vi "Dresden R2R Sputter 03.02.2018 IY24.vi"() -> ()   [LabVIEW 2009] (continued)
                      n14016 = case shown="False" w20577 {
                        tunnel: [FALSE ("Casette_servo_left_direction_do") TRUE ("Casette_servo_left_direction_do")] -> w20576
                        frame #0 {
                          n14017 = Wait Until Next ms Multiple(millisecond multiple=u32 200) -> ()  [unwired: 1 out]
                          n14018 = local write "Casette_servo_start/stop_do"(TRUE ("Casette_servo_left_direction_do")) -> ()
                        }
                        frame #1 {
                        }
                      }
                      n14019 = local read "Semi"() -> (w20575:bool)
                      n14020 = Or(x=w20576, y=w20575) -> (x .or. y?=w20574:bool)
                    }
                  }
                  frame #1 {
                    n14021 = local read "Semi"() -> (w20587:bool)
                    n14022 = case shown="False" w20587 {
                      frame #0 {
                        n14023 = local write "CH1_2trns_11"(TRUE ("CH1_2trns_9")) -> ()
                        n14024 = Wait (ms)(milliseconds to wait=u32 500) -> ()  [unwired: 1 out]
                      }
                      frame #1 {
                      }
                    }
                  }
                }
              }
              frame #1 {
              }
            }
          }
          frame #16 {
            # "Left sensors activate"
            n14025 = local read "Semi"() -> (w20590:bool)
            n14026 = case shown="False" w20590 {
              frame #0 {
                n14027 = stacked-sequence {
                  frame #0 {
                    n14028 = while {
                      i -> [w20599]
                      stop <- w20595 stop-if-true
                      n14029 = local read "Counter_read_data"() -> (w20592:i16)
                      n14030 = Greater?(x=w20599, y=1500) -> (0:w20598:bool)
                      n14031 = case shown="True" w20598 {
                        frame #0 {
                        }
                        frame #1 {
                          n14032 = local write "Semi"(TRUE ("Semi")) -> ()
                          n14033 = local write "Error Message"("Transfer process was cancelled.\nPlease check Casette & Sensor\nconnections." ("Error Message")) -> ()
                        }
                      }
                      n14034 = Greater Or Equal?(x=w20592, y=i16 5800) -> (x >= y?=w20593:bool)
                      n14035 = case shown="False" w20593 {
                        tunnel: [FALSE TRUE] -> w20596
                        frame #0 {
                          n14036 = Wait Until Next ms Multiple(millisecond multiple=u32 200) -> ()  [unwired: 1 out]
                        }
                        frame #1 {
                        }
                      }
                      n14037 = local read "Semi"() -> (w20594:bool)
                      n14038 = Or(x=w20596, y=w20594) -> (x .or. y?=w20595:bool)
                    }
                  }
                  frame #1 {
                    n14039 = while {
                      i -> [w20608]
                      stop <- w20605 stop-if-true
                      n14040 = Greater?(x=w20608, y=50) -> (0:w20609:bool)
                      n14041 = local read "Cnt_Left_slow_di"() -> (w20611:bool)
                      n14042 = case shown="True" w20609 {
                        frame #0 {
                        }
                        frame #1 {
                          n14043 = local write "Semi"(TRUE ("Semi")) -> ()
                          n14044 = local write "Error Message"("\nPlease check Left Slow Sensor\nconnections." ("Error Message")) -> ()
                        }
                      }
                      n14045 = case shown="True" w20611 {
                        tunnel: [TRUE ("Cnt_Left_slow_do") FALSE ("Cnt_Left_slow_do")] -> w20607
                        frame #0 {
                        }
                        frame #1 {
                          n14046 = Wait Until Next ms Multiple(millisecond multiple=u32 200) -> ()  [unwired: 1 out]
                          n14047 = local write "Cnt_Left_slow_do"(FALSE ("Cnt_Left_slow_do")) -> ()
                        }
                      }
                      n14048 = local read "Semi"() -> (w20606:bool)
                      n14049 = Or(x=w20607, y=w20606) -> (x .or. y?=w20605:bool)
                    }
                  }
                  frame #2 {
                    n14050 = while {
                      i -> [w20621]
                      stop <- w20618 stop-if-true
                      n14051 = Greater?(x=w20621, y=50) -> (0:w20622:bool)
                      n14052 = local read "Cnt_Left_limit_di"() -> (w20624:bool)
                      n14053 = case shown="True" w20622 {
                        frame #0 {
                        }
                        frame #1 {
                          n14054 = local write "Semi"(TRUE ("Semi")) -> ()
                          n14055 = local write "Error Message"("\nPlease check Left Limit Sensor\n connections." ("Error Message")) -> ()
                        }
                      }
                      n14056 = case shown="False" w20624 {
                        tunnel: [TRUE ("Cnt_Left_slow_do") FALSE ("Cnt_Left_slow_do")] -> w20620
                        frame #0 {
                        }
                        frame #1 {
                          n14057 = Wait Until Next ms Multiple(millisecond multiple=u32 200) -> ()  [unwired: 1 out]
                          n14058 = local write "Cnt_Left_limit_do"(FALSE ("Cnt_Left_slow_do")) -> ()
                        }
                      }
                      n14059 = local read "Semi"() -> (w20619:bool)
                      n14060 = Or(x=w20620, y=w20619) -> (x .or. y?=w20618:bool)
                    }
                  }
                  frame #3 {
                    n14061 = local read "Semi"() -> (w20631:bool)
                    n14062 = case shown="False" w20631 {
                      frame #0 {
                        n14063 = local write "CH1_2trns_12"(TRUE ("CH1_2trns_11")) -> ()
                        n14064 = Wait (ms)(milliseconds to wait=u32 500) -> ()  [unwired: 1 out]
                      }
                      frame #1 {
                      }
                    }
                  }
                }
              }
              frame #1 {
              }
            }
          }
          frame #17 {
            # "SET CASSETTE SERVO  SPEED 100"
            n14065 = local read "Semi"() -> (w20634:bool)
            n14066 = case shown="False" w20634 {
              frame #0 {
                n14067 = stacked-sequence {
                  frame #0 {
                    n14068 = while {
                      i -> [w20641]
                      stop <- w20637 stop-if-true
                      n14069 = local read "Ch4_Left_slow_di"() -> (w20635:bool)
                      n14070 = Greater?(x=w20641, y=1500) -> (0:w20640:bool)
                      n14071 = case shown="True" w20640 {
                        frame #0 {
                        }
                        frame #1 {
                          n14072 = local write "Semi"(TRUE ("Semi")) -> ()
                          n14073 = local write "Error Message"("Transfer process was cancelled.\nPlease check Casette & Sensor\nconnections." ("Error Message")) -> ()
                        }
                      }
                      n14074 = case shown="True" w20635 {
                        tunnel: [FALSE TRUE] -> w20638
                        frame #0 {
                          n14075 = Wait Until Next ms Multiple(millisecond multiple=u32 200) -> ()  [unwired: 1 out]
                        }
                        frame #1 {
                        }
                      }
                      n14076 = local read "Semi"() -> (w20636:bool)
                      n14077 = Or(x=w20638, y=w20636) -> (x .or. y?=w20637:bool)
                    }
                  }
                  frame #1 {
                    n14078 = disable-structure shown="Disabled" {
                      frame #0 {
                        n14079 = while {
                          i -> [w20656]
                          stop <- w20652 stop-if-true
                          n14080 = local read "Counter_read_data"() -> (w20649:i16)
                          n14081 = Greater?(x=w20656, y=5000) -> (0:w20655:bool)
                          n14082 = case shown="True" w20655 {
                            frame #0 {
                            }
                            frame #1 {
                              n14083 = local write "Semi"(TRUE ("Semi")) -> ()
                            }
                          }
                          n14084 = In Range and Coerce(upper limit=i16 1990, x=w20649, lower limit=i16 1980 ("upper limit")) -> (In Range?=w20647:bool)  [unwired: 1 out]
                          n14085 = case shown="True" w20647 {
                            tunnel: [FALSE TRUE] -> w20653
                            frame #0 {
                              n14086 = Wait Until Next ms Multiple(millisecond multiple=u32 200) -> ()  [unwired: 1 out]
                            }
                            frame #1 {
                            }
                          }
                          n14087 = local read "Semi"() -> (w20651:bool)
                          n14088 = Or(x=w20653, y=w20651) -> (x .or. y?=w20652:bool)
                        }
                      }
                      frame #1 {
                      }
                    }
                  }
                  frame #2 {
                    n14089 = local read "Semi"() -> (w20661:bool)
                    n14090 = case shown="False" w20661 {
                      frame #0 {
                        n14091 = local write "Cassette_servo_speed_value"(u16 100 ("Cassette_servo_speed_value")) -> ()
                      }
                      frame #1 {
                      }
                    }
                  }
                  frame #3 {
                    n14092 = local read "Semi"() -> (w20663:bool)
                    n14093 = case shown="False" w20663 {
                      frame #0 {
                        n14094 = Wait (ms)(milliseconds to wait=u32 200 ("millisecond multiple")) -> ()  [unwired: 1 out]
                      }
                      frame #1 {
                      }
                    }
                  }
                  frame #4 {
                    n14095 = local read "Semi"() -> (w20665:bool)
                    n14096 = case shown="False" w20665 {
                      frame #0 {
                        n14097 = local write "Cassette_servo_speed_auto_set"(TRUE ("Cassette_servo_speed_auto_set")) -> ()
                      }
                      frame #1 {
                      }
                    }
                  }
                  frame #5 {
                    n14098 = local read "Semi"() -> (w20667:bool)
                    n14099 = case shown="False" w20667 {
                      frame #0 {
                        n14100 = Wait (ms)(milliseconds to wait=u32 200 ("millisecond multiple")) -> ()  [unwired: 1 out]
                      }
                      frame #1 {
                      }
                    }
                  }
                  frame #6 {
                    n14101 = while {
                      i -> [w20672]
                      stop <- w20669 stop-if-true
                      n14102 = Greater?(x=w20672, y=50) -> (0:w20673:bool)
                      n14103 = local read "Cnt_Left_slow_di"() -> (w20675:bool)
                      n14104 = case shown="True" w20673 {
                        frame #0 {
                        }
                        frame #1 {
                          n14105 = local write "Semi"(TRUE ("Semi")) -> ()
                          n14106 = local write "Error Message"("\nPlease check connections." ("Error Message")) -> ()
                        }
                      }
                      n14107 = case shown="False" w20675 {
                        tunnel: [FALSE ("Cnt_Left_slow_do") TRUE ("Cnt_Left_slow_do")] -> w20671
                        frame #0 {
                          n14108 = Wait Until Next ms Multiple(millisecond multiple=u32 200) -> ()  [unwired: 1 out]
                          n14109 = local write "Cnt_Left_slow_do"(TRUE ("Cnt_Left_slow_do")) -> ()
                        }
                        frame #1 {
                        }
                      }
                      n14110 = local read "Semi"() -> (w20670:bool)
                      n14111 = Or(x=w20671, y=w20670) -> (x .or. y?=w20669:bool)
                    }
                  }
                  frame #7 {
                    n14112 = local read "Semi"() -> (w20682:bool)
                    n14113 = case shown="False" w20682 {
                      frame #0 {
                        n14114 = local write "CH1_2trns_12"(TRUE ("CH1_2trns_11")) -> ()
                        n14115 = Wait (ms)(milliseconds to wait=u32 500) -> ()  [unwired: 1 out]
                      }
                      frame #1 {
                      }
                    }
                  }
                }
              }
              frame #1 {
              }
            }
          }
          frame #18 {
            # "CASETTE STOP AND FIX"
            n14116 = local read "Semi"() -> (w20685:bool)
            n14117 = case shown="False" w20685 {
              frame #0 {
                n14118 = stacked-sequence {
                  frame #0 {
                    # "Center Casette stop"
                    n14119 = local read "Semi"() -> (w20686:bool)
                    n14120 = case shown="False" w20686 {
                      frame #0 {
                        n14121 = stacked-sequence {
                          frame #0 {
                            n14122 = while {
                              i -> [w20693]
                              stop <- w20688 stop-if-true
                              n14123 = local read "Ch4_Left_limit_di"() -> (w20687:bool)
                              n14124 = Greater?(x=w20693, y=600) -> (0:w20691:bool)
                              n14125 = case shown="True" w20691 {
                                frame #0 {
                                }
                                frame #1 {
                                n14126 = local write "Semi"(TRUE ("Semi")) -> ()
                                n14127 = local write "Error Message"("Transfer process was cancelled.\nPlease check Casette connections." ("Error Message")) -> ()
                                }
                              }
                              n14128 = case shown="False" w20687 {
                                tunnel: [FALSE TRUE] -> w20690
                                frame #0 {
                                n14129 = Wait Until Next ms Multiple(millisecond multiple=u32 200) -> ()  [unwired: 1 out]
                                }
                                frame #1 {
                                }
                              }
                              n14130 = local read "Semi"() -> (w20689:bool)
                              n14131 = Or(x=w20690, y=w20689) -> (x .or. y?=w20688:bool)
                            }
                          }
                          frame #1 {
                            n14132 = disable-structure shown="Disabled" {
                              frame #0 {
                                n14133 = while {
                                i -> [w20708]
                                stop <- w20703 stop-if-true
                                n14134 = local read "Counter_read_data"() -> (w20700:i16)
                                n14135 = Greater?(x=w20708, y=5000) -> (0:w20706:bool)
                                n14136 = case shown="True" w20706 {
                                frame #0 {
                                }
                                frame #1 {
                                n14137 = local write "Semi"(TRUE ("Semi")) -> ()
                                n14138 = local write "Error Message"("Transfer process was cancelled.\nPlease check Casette connections." ("Error Message")) -> ()
                                }
                                }
                                n14139 = In Range and Coerce(upper limit=i16 2209, x=w20700, lower limit=i16 2199 ("upper limit")) -> (In Range?=w20699:bool)  [unwired: 1 out]
                                n14140 = case shown="True" w20699 {
                                tunnel: [FALSE TRUE] -> w20705
                                frame #0 {
                                }
                                frame #1 {
                                n14141 = Wait Until Next ms Multiple(millisecond multiple=u32 500) -> ()  [unwired: 1 out]
                                }
                                }
                                n14142 = local read "Semi"() -> (w20704:bool)
                                n14143 = Or(x=w20705, y=w20704) -> (x .or. y?=w20703:bool)
                                }
                              }
                              frame #1 {
                              }
                            }
                          }
                          frame #2 {
                            n14144 = while {
                              i -> [w20720]
                              stop <- w20715 stop-if-true
                              n14145 = local read "Casette_servo_start/stop_di"() -> (w20714:bool)
                              n14146 = Greater?(x=w20720, y=50) -> (0:w20718:bool)
                              n14147 = case shown="True" w20718 {
                                frame #0 {
                                }
                                frame #1 {
                                n14148 = local write "Semi"(TRUE ("Semi")) -> ()
                                n14149 = local write "Error Message"("Transfer process was cancelled.\nPlease check Casette connections." ("Error Message")) -> ()
                                }
                              }
                              n14150 = case shown="True" w20714 {
                                tunnel: [TRUE FALSE] -> w20717
                                frame #0 {
                                }
                                frame #1 {
                                n14151 = Wait Until Next ms Multiple(millisecond multiple=u32 200) -> ()  [unwired: 1 out]
                                n14152 = local write "Casette_servo_start/stop_do"(FALSE ("Casette_servo_start/stop_di")) -> ()
                                }
                              }
                              n14153 = local read "Semi"() -> (w20716:bool)
                              n14154 = Or(x=w20717, y=w20716) -> (x .or. y?=w20715:bool)
                            }
                          }
                          frame #3 {
                            n14155 = local read "Semi"() -> (w20727:bool)
                            n14156 = case shown="False" w20727 {
                              frame #0 {
                                n14157 = Wait (ms)(milliseconds to wait=u32 200) -> ()  [unwired: 1 out]
                              }
                              frame #1 {
                              }
                            }
                          }
                          frame #4 {
                            n14158 = local read "Semi"() -> (w20729:bool)
                            n14159 = case shown="False" w20729 {
                              frame #0 {
                                n14160 = local write "Cassette_servo_speed_value"(u16 0 ("Cassette_servo_speed_value")) -> ()
                              }
                              frame #1 {
                              }
                            }
                          }
                          frame #5 {
                            n14161 = local read "Semi"() -> (w20731:bool)
                            n14162 = case shown="False" w20731 {
                              frame #0 {
                                n14163 = Wait (ms)(milliseconds to wait=u32 200) -> ()  [unwired: 1 out]
                              }
                              frame #1 {
                              }
                            }
                          }
                          frame #6 {
                            n14164 = local read "Semi"() -> (w20733:bool)
                            n14165 = case shown="False" w20733 {
                              frame #0 {
                                n14166 = local write "Cassette_servo_speed_auto_set"(TRUE ("Cassette_servo_speed_auto_set")) -> ()
                              }
                              frame #1 {
                              }
                            }
                          }
                          frame #7 {
                            n14167 = local read "Semi"() -> (w20735:bool)
                            n14168 = case shown="False" w20735 {
                              frame #0 {
                                n14169 = Wait (ms)(milliseconds to wait=u32 200) -> ()  [unwired: 1 out]
                              }
                              frame #1 {
                              }
                            }
                          }
                          frame #8 {
                            n14170 = local read "Semi"() -> (w20737:bool)
                            n14171 = case shown="False" w20737 {
                              frame #0 {
                                n14172 = local write "CH1_2trns_13"(TRUE ("CH1_2trns_9")) -> ()
                                n14173 = Wait (ms)(milliseconds to wait=u32 500) -> ()  [unwired: 1 out]
                              }
                              frame #1 {
                              }
                            }
                          }
                        }
                      }
                      frame #1 {
                      }
                    }
                  }
                  frame #1 {
                    # "CASETTE FIX DOWN CH2"
                    n14174 = local read "Semi"() -> (w20740:bool)
                    n14175 = case shown="False" w20740 {
                      frame #0 {
                        n14176 = stacked-sequence {
                          frame #0 {
                            n14177 = local read "Semi"() -> (w20741:bool)
                            n14178 = case shown="False" w20741 {
                              frame #0 {
                                n14179 = while {
                                i -> [w20748]
                                stop <- w20743 stop-if-true
                                n14180 = Greater?(x=w20748, y=50) -> (0:w20746:bool)
                                n14181 = local read "Ch4_Cst_fix_down_di"() -> (w20742:bool)
                                n14182 = case shown="True" w20746 {
                                frame #0 {
                                }
                                frame #1 {
                                n14183 = local write "Semi"(TRUE ("Semi")) -> ()
                                n14184 = local write "Error Message"("Up/Down positions could not reach\nthe down position.\nPlease check connections." ("Error Message")) -> ()
                                }
                                }
                                n14185 = case shown="False" w20742 {
                                tunnel: [FALSE TRUE] -> w20745
                                frame #0 {
                                n14186 = Wait Until Next ms Multiple(millisecond multiple=u32 200) -> ()  [unwired: 1 out]
                                n14187 = local write "Ch4_Cst_fix_do"(TRUE ("Ch1_pet_cool_up_do")) -> ()
                                }
                                frame #1 {
                                }
                                }
                                n14188 = local read "Semi"() -> (w20744:bool)
                                n14189 = Or(x=w20745, y=w20744) -> (x .or. y?=w20743:bool)
                                }
                              }
                              frame #1 {
                              }
                            }
                          }
                          frame #1 {
                            n14190 = local read "Semi"() -> (w20755:bool)
                            n14191 = case shown="False" w20755 {
                              frame #0 {
                                n14192 = local write "CH1_2trns_14"(TRUE ("CH1_2trns_9")) -> ()
                                n14193 = Wait (ms)(milliseconds to wait=u32 500) -> ()  [unwired: 1 out]
                              }
                              frame #1 {
                              }
                            }
                          }
                        }
                      }
                      frame #1 {
                      }
                    }
                  }
                  frame #2 {
                    n14194 = local read "Semi"() -> (w20758:bool)
                    n14195 = case shown="False" w20758 {
                      frame #0 {
                        n14196 = stacked-sequence {
                          frame #0 {
                            n14197 = local read "Semi"() -> (w20759:bool)
                            n14198 = case shown="False" w20759 {
                              frame #0 {
                                n14199 = while {
                                i -> [w20766]
                                stop <- w20761 stop-if-true
                                n14200 = Greater?(x=w20766, y=50) -> (0:w20764:bool)
                                n14201 = local read "Ch4_Trns_gv_bp_di"() -> (w20760:bool)
                                n14202 = case shown="True" w20764 {
                                frame #0 {
                                }
                                frame #1 {
                                n14203 = local write "Semi"(TRUE ("Semi")) -> ()
                                n14204 = local write "Error Message"("Transfer process was cancelled.\nPlease check CH1-Trns-GV connections." ("Error Message")) -> ()
                                }
                                }
                                n14205 = case shown="True" w20760 {
                                tunnel: [TRUE FALSE] -> w20763
                                frame #0 {
                                }
                                frame #1 {
                                n14206 = Wait Until Next ms Multiple(millisecond multiple=u32 200) -> ()  [unwired: 1 out]
                                n14207 = local write "Ch4_Trns_gv_bp_do"(FALSE ("Ch1_pet_cool_up_do")) -> ()
                                }
                                }
                                n14208 = local read "Semi"() -> (w20762:bool)
                                n14209 = Or(x=w20763, y=w20762) -> (x .or. y?=w20761:bool)
                                }
                              }
                              frame #1 {
                              }
                            }
                          }
                          frame #1 {
                            n14210 = local read "Semi"() -> (w20773:bool)
                            n14211 = case shown="False" w20773 {
                              frame #0 {
                                n14212 = Wait (ms)(milliseconds to wait=u32 500) -> ()  [unwired: 1 out]
                              }
                              frame #1 {
                              }
                            }
                          }
                          frame #2 {
                            n14213 = local read "Semi"() -> (w20775:bool)
                            n14214 = case shown="False" w20775 {
                              frame #0 {
                                n14215 = while {
                                i -> [w20782]
                                stop <- w20777 stop-if-true
                                n14216 = Greater?(x=w20782, y=50) -> (0:w20780:bool)
                                n14217 = local read "Ch3_Trns_gv_bp2_di"() -> (w20776:bool)
                                n14218 = case shown="True" w20780 {
                                frame #0 {
                                }
                                frame #1 {
                                n14219 = local write "Semi"(TRUE ("Semi")) -> ()
                                n14220 = local write "Error Message"("Transfer process was cancelled.\nPlease check CH1-Trns-GV connections." ("Error Message")) -> ()
                                }
                                }
                                n14221 = case shown="True" w20776 {
                                tunnel: [TRUE FALSE] -> w20779
                                frame #0 {
                                }
                                frame #1 {
                                n14222 = local write "Ch3_Trns_gv_bp2_do"(FALSE ("Ch1_pet_cool_up_do")) -> ()
                                n14223 = Wait Until Next ms Multiple(millisecond multiple=u32 200) -> ()  [unwired: 1 out]
                                }
                                }
                                n14224 = local read "Semi"() -> (w20778:bool)
                                n14225 = Or(x=w20779, y=w20778) -> (x .or. y?=w20777:bool)
                                }
                              }
                              frame #1 {
                              }
                            }
                          }
                          frame #3 {
                            n14226 = local read "Semi"() -> (w20789:bool)
                            n14227 = case shown="False" w20789 {
                              frame #0 {
                                n14228 = Wait (ms)(milliseconds to wait=u32 500) -> ()  [unwired: 1 out]
                              }
                              frame #1 {
                              }
                            }
                          }
                        }
                      }
                      frame #1 {
                      }
                    }
                  }
                  frame #3 {
                    n14229 = local read "Semi"() -> (w20791:bool)
                    n14230 = case shown="False" w20791 {
                      frame #0 {
                        n14231 = stacked-sequence {
                          frame #0 {
                            n14232 = local read "Semi"() -> (w20792:bool)
                            n14233 = case shown="False" w20792 {
                              frame #0 {
                                n14234 = local write "Ch3_Trns_gv_open_do"(FALSE ("Ch1_pet_cool_up_do")) -> ()
                              }
                              frame #1 {
                              }
                            }
                          }
                          frame #1 {
                            n14235 = local read "Semi"() -> (w20794:bool)
                            n14236 = case shown="False" w20794 {
                              frame #0 {
                                n14237 = while {
                                i -> [w20801]
                                stop <- w20796 stop-if-true
                                n14238 = Greater?(x=w20801, y=500) -> (0:w20799:bool)
                                n14239 = local read "Ch3_Trns_gv_close_di"() -> (w20795:bool)
                                n14240 = case shown="True" w20799 {
                                frame #0 {
                                }
                                frame #1 {
                                n14241 = local write "Semi"(TRUE ("Semi")) -> ()
                                n14242 = local write "Error Message"("Transfer process was cancelled.\nPlease check  GV connections." ("Error Message")) -> ()
                                }
                                }
                                n14243 = case shown="False" w20795 {
                                tunnel: [FALSE TRUE] -> w20798
                                frame #0 {
                                n14244 = Wait Until Next ms Multiple(millisecond multiple=u32 200) -> ()  [unwired: 1 out]
                                n14245 = local write "Ch3_Trns_gv_close_do"(TRUE ("Ch1_pet_cool_up_do")) -> ()
                                }
                                frame #1 {
                                }
                                }
                                n14246 = local read "Semi"() -> (w20797:bool)
                                n14247 = Or(x=w20798, y=w20797) -> (x .or. y?=w20796:bool)
                                }
                              }
                              frame #1 {
                              }
                            }
                          }
                          frame #2 {
                            n14248 = local read "Semi"() -> (w20808:bool)
                            n14249 = case shown="False" w20808 {
                              frame #0 {
                                n14250 = local write "CH1_2trns_17"(TRUE ("CH1_2trns_9")) -> ()
                                n14251 = Wait (ms)(milliseconds to wait=u32 500) -> ()  [unwired: 1 out]
                              }
                              frame #1 {
                              }
                            }
                          }
                        }
                      }
                      frame #1 {
                      }
                    }
                  }
                  frame #4 {
                    # "PET COOL DOWN OF CH2"
                    n14252 = local read "Semi"() -> (w20811:bool)
                    n14253 = case shown="False" w20811 {
                      frame #0 {
                        n14254 = stacked-sequence {
                          frame #0 {
                            n14255 = local read "Semi"() -> (w20812:bool)
                            n14256 = case shown="False" w20812 {
                              frame #0 {
                                n14257 = local write "Ch4_Pet_cool_up_do"(FALSE ("Ch1_pet_cool_up_do")) -> ()
                              }
                              frame #1 {
                              }
                            }
                          }
                          frame #1 {
                            n14258 = local read "Semi"() -> (w20814:bool)
                            n14259 = case shown="False" w20814 {
                              frame #0 {
                                n14260 = while {
                                i -> [w20821]
                                stop <- w20816 stop-if-true
                                n14261 = Greater?(x=w20821, y=300) -> (0:w20819:bool)
                                n14262 = case shown="True" w20819 {
                                frame #0 {
                                }
                                frame #1 {
                                n14263 = local write "Semi"(TRUE ("Semi")) -> ()
                                n14264 = local write "Error Message"("SBS Cool Up/Down positions could not reach\nthe down position.\nPlease check connections." ("Error Message")) -> ()
                                }
                                }
                                n14265 = local read "Ch4_Pet_cool_down_di"() -> (w20815:bool)
                                n14266 = case shown="False" w20815 {
                                tunnel: [FALSE TRUE] -> w20818
                                frame #0 {
                                n14267 = Wait Until Next ms Multiple(millisecond multiple=u32 200) -> ()  [unwired: 1 out]
                                n14268 = local write "Ch4_Pet_cool_down_do"(TRUE ("Ch1_pet_cool_up_do")) -> ()
                                }
                                frame #1 {
                                }
                                }
                                n14269 = local read "Semi"() -> (w20817:bool)
                                n14270 = Or(x=w20818, y=w20817) -> (x .or. y?=w20816:bool)
                                }
                              }
                              frame #1 {
                              }
                            }
                          }
                          frame #2 {
                            n14271 = local read "Semi"() -> (w20828:bool)
                            n14272 = case shown="False" w20828 {
                              frame #0 {
                                n14273 = local write "CH1_2trns_15"(TRUE ("CH1_2trns_9")) -> ()
                                n14274 = Wait (ms)(milliseconds to wait=u32 500) -> ()  [unwired: 1 out]
                              }
                              frame #1 {
                              }
                            }
                          }
                        }
                      }
                      frame #1 {
                      }
                    }
                  }
                  frame #5 {
                    # "SRV PIS FOR"
                    n14275 = local read "Semi"() -> (w20831:bool)
                    n14276 = case shown="False" w20831 {
                      frame #0 {
                        n14277 = stacked-sequence {
                          frame #0 {
                            n14278 = local read "Semi"() -> (w20832:bool)
                            n14279 = case shown="False" w20832 {
                              frame #0 {
                                n14280 = local write "Ch4_SRV1_PIST_Back_do"(FALSE ("Ch1_pet_cool_up_do")) -> ()
                              }
                              frame #1 {
                              }
                            }
                          }
                          frame #1 {
                            n14281 = local read "Semi"() -> (w20834:bool)
                            n14282 = case shown="False" w20834 {
                              frame #0 {
                                n14283 = while {
                                i -> [w20841]
                                stop <- w20836 stop-if-true
                                n14284 = Greater?(x=w20841, y=100) -> (0:w20839:bool)
                                n14285 = local read "Ch4_SRV1_PIST For_di"() -> (w20835:bool)
                                n14286 = case shown="True" w20839 {
                                frame #0 {
                                }
                                frame #1 {
                                n14287 = local write "Semi"(TRUE ("Semi")) -> ()
                                n14288 = local write "Error Message"("For/Back positions could not reach\nthe forward position.\nPlease check connections." ("Error Message")) -> ()
                                }
                                }
                                n14289 = case shown="False" w20835 {
                                tunnel: [FALSE TRUE] -> w20838
                                frame #0 {
                                n14290 = Wait Until Next ms Multiple(millisecond multiple=u32 200) -> ()  [unwired: 1 out]
                                n14291 = local write "Ch4_SRV1_PIST For_do"(TRUE ("Ch1_pet_cool_up_do")) -> ()
                                }
                                frame #1 {
                                }
                                }
                                n14292 = local read "Semi"() -> (w20837:bool)
                                n14293 = Or(x=w20838, y=w20837) -> (x .or. y?=w20836:bool)
                                }
                              }
                              frame #1 {
                              }
                            }
                          }
                          frame #2 {
                            n14294 = local read "Semi"() -> (w20848:bool)
                            n14295 = case shown="False" w20848 {
                              frame #0 {
                                n14296 = local write "CH1_2trns_16"(TRUE ("CH1_2trns_9")) -> ()
                                n14297 = Wait (ms)(milliseconds to wait=u32 500) -> ()  [unwired: 1 out]
                              }
                              frame #1 {
                              }
                            }
                          }
                        }
                      }
                      frame #1 {
                      }
                    }
                  }
                }
              }
              frame #1 {
              }
            }
          }
          frame #19 {
            # "Sensors deactive"
            n14298 = local read "Semi"() -> (w20851:bool)
            n14299 = case shown="False" w20851 {
              frame #0 {
                n14300 = stacked-sequence {
                  frame #0 {
                    n14301 = local read "Semi"() -> (w20852:bool)
                    n14302 = case shown="False" w20852 {
                      frame #0 {
                        n14303 = while {
                          i -> [w20855]
                          stop <- w20856 stop-if-true
                          n14304 = Greater?(x=w20855, y=50) -> (0:w20853:bool)
                          n14305 = local read "Cnt_Right_slow_di"() -> (w20859:bool)
                          n14306 = case shown="True" w20853 {
                            frame #0 {
                            }
                            frame #1 {
                              n14307 = local write "Semi"(TRUE ("Semi")) -> ()
                              n14308 = local write "Error Message"("Transfer process was\ncancelled.Please check right slow sensor." ("Error Message")) -> ()
                            }
                          }
                          n14309 = case shown="False" w20859 {
                            tunnel: [FALSE ("Ch1_pet_cool_up_do") TRUE ("Ch1_pet_cool_up_do")] -> w20858
                            frame #0 {
                              n14310 = Wait Until Next ms Multiple(millisecond multiple=u32 200) -> ()  [unwired: 1 out]
                              n14311 = local write "Cnt_Right_slow_do"(TRUE ("Ch1_pet_cool_up_do")) -> ()
                            }
                            frame #1 {
                            }
                          }
                          n14312 = local read "Semi"() -> (w20857:bool)
                          n14313 = Or(x=w20858, y=w20857) -> (x .or. y?=w20856:bool)
                        }
                      }
                      frame #1 {
                      }
                    }
                  }
                  frame #1 {
                    n14314 = local read "Semi"() -> (w20866:bool)
                    n14315 = case shown="False" w20866 {
                      frame #0 {
                        n14316 = while {
                          i -> [w20869]
                          stop <- w20870 stop-if-true
                          n14317 = Greater?(x=w20869, y=50) -> (0:w20867:bool)
                          n14318 = local read "Cnt_Right_limit_di"() -> (w20873:bool)
                          n14319 = case shown="True" w20867 {
                            frame #0 {
                            }
                            frame #1 {
                              n14320 = local write "Semi"(TRUE ("Semi")) -> ()
                              n14321 = local write "Error Message"("Transfer process was\ncancelled.Please check right limit sensor." ("Error Message")) -> ()
                            }
                          }
                          n14322 = case shown="False" w20873 {
                            tunnel: [FALSE ("Ch1_pet_cool_up_do") TRUE ("Ch1_pet_cool_up_do")] -> w20872
                            frame #0 {
                              n14323 = Wait Until Next ms Multiple(millisecond multiple=u32 200) -> ()  [unwired: 1 out]
                              n14324 = local write "Cnt_Right_limit_do"(TRUE ("Ch1_pet_cool_up_do")) -> ()
                            }
                            frame #1 {
                            }
                          }
                          n14325 = local read "Semi"() -> (w20871:bool)
                          n14326 = Or(x=w20872, y=w20871) -> (x .or. y?=w20870:bool)
                        }
                      }
                      frame #1 {
                      }
                    }
                  }
                  frame #2 {
                    n14327 = local read "Semi"() -> (w20880:bool)
                    n14328 = case shown="False" w20880 {
                      frame #0 {